vi "15-12-13 UHR-Fleezers Control (host) - 15.2.1UCB Darwin.vi"() -> ()   [LabVIEW 2014] (continued)
    n2915 = Build Array(w4201, w4200) -> (w4199:dbl[][])
    n2916 = Bundle(w4053, w4052, w4002) -> (w4057:cluster{u32[], u32[], u32[]})  [unwired: 1 in]
    n2917 = Build Array(w4053, w4052, w4002) -> (w4297:u32[][])
    n2918 = for {
      tunnel: w4053 -> [w4445] mode=indexing
      n2919 = call "Smart Buffer (DBL) 1.vi"("new element [write]"=w4445, "mode"=T25."write") -> ()  [unwired: 4 in, 6 out]
    }
    n2920 = local read "APD Integration Time (s)"() -> (w4068:dbl)
    n2921 = To Double Precision Float(number=w4297) -> (double precision float=w4298:dbl[][])
    n2922 = feedback #7 "APD3"(w4002) -> (w4003:u32[])
    n2923 = feedback #8 "APD2"(w4052) -> (w4225:u32[])
    n2924 = feedback #9 "APD1"(w4053) -> (w4296:u32[])
    n2925 = Build Array (concatenate)(w4003, w4002) -> (w4001:u32[])
    n2926 = Build Array (concatenate)(w4225, w4052) -> (w4224:u32[])
    n2927 = Build Array (concatenate)(w4296, w4053) -> (w4293:u32[])
    n2928 = for {
      tunnel: w4052 -> [w4444] mode=indexing
      n2929 = call "Smart Buffer (DBL) 2.vi"("new element [write]"=w4444, "mode"=T25."write") -> ()  [unwired: 4 in, 6 out]
    }
    n2930 = Array Size(array=w4293) -> (size(s)=w4290:i32)
    n2931 = Array Size(array=w4053) -> (size(s)=w4292:i32)
    n2932 = Multiply(x=w4292, y="APD Ave N") -> (x*y=w4291:dbl)
    n2933 = Greater?(x=w4290, y=w4291) -> (0:w4294:bool)
    n2934 = Bundle("APD 1", "APD 2", "APD 3") -> (w4328:cluster{string, string, string})  [unwired: 1 out]
    n2935 = local read "Trap Sets"() -> (w4260:u32)
    n2936 = case shown="True" w4294 {
      tunnel: w4293 -> [w4701 w4710]
      tunnel: [w4701 w4708] -> w4267
      tunnel: w4291 -> [_ w4703]
      tunnel: w4290 -> [_ w4709]
      tunnel: w4224 -> [w4700 w4707]
      tunnel: [w4700 w4706] -> w4222
      tunnel: w4001 -> [w4699 w4705]
      tunnel: [w4699 w4702] -> w4069
      frame False {
      }
      frame True {
        n2937 = Subtract(x=w4709, y=w4703) -> (x-y=w4704:dbl)
        n2938 = Array Subset "APD3"(array=w4705, index=w4704, length=w4703) -> (w4702:u32[])
        n2939 = Array Subset "APD2"(array=w4707, index=w4704, length=w4703) -> (w4706:u32[])
        n2940 = Array Subset "APD1"(array=w4710, index=w4704, length=w4703) -> (w4708:u32[])
      }
    }
    n2941 = feedback-in #7(w4069) -> ()
    n2942 = feedback-in #8(w4222) -> ()
    n2943 = feedback-in #9(w4267) -> ()
    n2944 = Cluster To Array(cluster=w4328) -> (array=w4325:string[])
    n2945 = for "APD" {
      tunnel: w4298 -> [w4970] mode=indexing
      tunnel: w4068 -> [w4977]
      tunnel: [w4973] -> w4226 mode=indexing
      tunnel: "APD Disp. Scale" -> [w4974]
      tunnel: w4325 -> [w4972] mode=indexing
      tunnel: "APD Disp. Downsample" -> [w4968]
      tunnel: [w4971] -> w4324
      workers-P: _ -> [_]
      tunnel: w4195 -> [w4967]
      n2946 = call "integrate 1D array interval - double.vi"("Ave N"=w4968, "Array In"=w4970) -> ("Array Out"=w4969:dbl[])  [unwired: 1 out]
      n2947 = Multiply(x=w4977, y=w4968) -> (x*y=w4971:dbl)
      n2948 = Divide(x=w4969, y=w4974) -> (x/y=w4975:dbl[])
      n2949 = Bundle By Name("t0"=w4967, "Y"=w4975, "dt"=w4971) -> (w4976:waveform(dbl))  [unwired: 1 out]
      n2950 = Set Waveform Attribute(5:w4972, 6:"NI_ChannelName" ("name"), 7:w4976) -> (3:w4973:waveform(dbl))  [unwired: 1 in, 2 out]
    }
    "APD Display Period (s)" <- w4324
    n2951 = Reciprocal(x=w4324) -> (1/x=→"APD Display Freq. (Hz)":dbl)
    n2952 = case "Deinterlace trap data, average down PSD" shown="2" w4260 {
      tunnel: w4168 -> [w4995 w5060]
      tunnel: [w4992 w5057] -> w4255
      tunnel: [w4995 w5059] -> w4159
      tunnel: "Detector Type" -> [w4994 w5055]
      tunnel: [w4993 w5058] -> w4254
      tunnel: [w4991 w5056] -> w4332
      frame 1, Default {
        n2953 = Divide(x=w4995, y=3276.7) -> (x/y=w4996:dbl[])
        n2954 = Decimate 1D Array(w4996) -> (w5005:dbl[], w5004:dbl[], w5003:dbl[], w5002:dbl[], w5001:dbl[], w5000:dbl[], w4999:dbl[], w4998:dbl[])
        n2955 = case shown="\"IR-QPD + PSD + FB-QPD position\"" w4994 {
          tunnel: w5005 -> [w5029 w5054]
          tunnel: w5004 -> [w5028 w5053]
          tunnel: w5003 -> [w5013 w5031]
          tunnel: w5002 -> [w5014 w5041]
          tunnel: w5001 -> [w5027 w5052]
          tunnel: w5000 -> [w5026 w5051]
          tunnel: w4999 -> [w5010 w5032]
          tunnel: w4998 -> [w5009 w5030]
          tunnel: [w5008 w5038] -> w4993
          tunnel: [w5007 w5037] -> w4992
          tunnel: [w5006 w5036] -> w4991
          frame "IR-QPD + PSD + FB-QPD", Default {
            w5006 = 0  # Channel pattern
            n2956 = Divide(x=w5029, y=w5014) -> (x/y=w5016:dbl[])
            n2957 = Divide(x=w5028, y=w5014) -> (x/y=w5015:dbl[])
            n2958 = Divide(x=w5027, y=w5010) -> (x/y=w5012:dbl[])
            n2959 = Divide(x=w5026, y=w5009) -> (x/y=w5011:dbl[])
            n2960 = Build Array(w5016, w5015, w5014, w5013, w5012, w5011, w5010, w5009) -> (w5007:dbl[][])
            n2961 = Bundle("T1 Y", "T1 X", "T1 Sum", "FB Sum", "PSD Y", "PSD X", "PSD Y Sum", "PSD X Sum") -> (w5025:T49)  [unwired: 1 out]
            n2962 = Cluster To Array(cluster=w5025) -> (array=w5008:string[])
          }
          frame "IR-QPD + PSD + FB-QPD position" {
            w5036 = 3  # Channel pattern
            n2963 = Negate(x=w5032) -> (-x=w5033:dbl[])
            n2964 = Divide(x=w5054, y=w5041) -> (x/y=w5043:dbl[])
            n2965 = Divide(x=w5053, y=w5041) -> (x/y=w5042:dbl[])
            n2966 = Divide(x=w5052, y=w5032) -> (x/y=w5040:dbl[])
            n2967 = Divide(x=w5051, y=w5033) -> (x/y=w5039:dbl[])
            n2968 = Build Array(w5043, w5042, w5041, w5030, w5031, w5040, w5039, w5032) -> (w5037:dbl[][])
            n2969 = Bundle("T1 Y", "T1 X", "T1 Sum", "FB X", "FB Sum", "PSD Y", "PSD X", "PSD Y Sum") -> (w5050:T49)  [unwired: 1 out]
            n2970 = Cluster To Array(cluster=w5050) -> (array=w5038:string[])
          }
        }
      }
      frame 2 {
        n2971 = case shown="\"IR-QPD + PSD + FB-QPD X position\", Default" w5055 {
          tunnel: w5060 -> [w5122 w5194 w5265]
          tunnel: [w5061 w5185 w5196] -> w5059
          tunnel: [w5088 w5176 w5243] -> w5058
          tunnel: [w5087 w5139 w5210] -> w5057
          tunnel: [w5081 w5174 w5241] -> w5056
          frame "IR-QPD + PSD + FB-QPD" {
            w5081 = 1  # Channel pattern
            # "time average x2 the 4th signal and the 4 psd signals (detection laser)"
            # "deinterlace 3 signals from qpd"
            n2972 = Decimate 1D Array(w5122) -> (w5121:i16[], w5120:i16[], w5086:i16[], w5119:i16[], w5109:i16[], w5107:i16[], w5106:i16[], w5104:i16[])
            n2973 = Decimate 1D Array(w5086) -> (w5085:i16[], w5084:i16[])
            n2974 = Decimate 1D Array(w5121) -> (w5118:i16[], w5090:i16[])
            n2975 = Decimate 1D Array(w5120) -> (w5117:i16[], w5115:i16[])
            n2976 = Decimate 1D Array(w5119) -> (w5116:i16[], w5114:i16[])
            n2977 = call "downsample 1D array - double.vi"("Ave N"=2.0, "Array In"=w5109) -> ("Array Out"=w5108:dbl[])  [unwired: 1 out]
            n2978 = call "downsample 1D array - double.vi"("Ave N"=2.0, "Array In"=w5107) -> ("Array Out"=w5089:dbl[])  [unwired: 1 out]
            n2979 = call "downsample 1D array - double.vi"("Ave N"=2.0, "Array In"=w5106) -> ("Array Out"=w5105:dbl[])  [unwired: 1 out]
            n2980 = call "downsample 1D array - double.vi"("Ave N"=2.0, "Array In"=w5104) -> ("Array Out"=w5103:dbl[])  [unwired: 1 out]
            n2981 = Interleave 1D Arrays(w5118, w5117, w5116, w5090, w5115, w5114, w5085, w5084, w5108, w5089, w5105, w5103) -> (w5102:dbl[])
            n2982 = Divide(x=w5102, y=3276.7) -> (x/y=w5101:dbl[])
            n2983 = Decimate 1D Array(w5101) -> (w5100:dbl[], w5099:dbl[], w5098:dbl[], w5097:dbl[], w5096:dbl[], w5095:dbl[], w5083:dbl[], w5082:dbl[], w5094:dbl[], w5093:dbl[], w5092:dbl[], w5091:dbl[])
            n2984 = Divide(x=w5100, y=w5098) -> (x/y=w5068:dbl[])
            n2985 = Divide(x=w5099, y=w5098) -> (x/y=w5067:dbl[])
            n2986 = Divide(x=w5097, y=w5095) -> (x/y=w5066:dbl[])
            n2987 = Divide(x=w5096, y=w5095) -> (x/y=w5065:dbl[])
            n2988 = Divide(x=w5094, y=w5092) -> (x/y=w5064:dbl[])
            n2989 = Divide(x=w5093, y=w5091) -> (x/y=w5063:dbl[])
            n2990 = Build Array(w5068, w5067, w5098, w5066, w5065, w5095, w5083, w5082, w5064, w5063, w5092, w5091) -> (w5087:dbl[][])
            n2991 = Bundle("T1 Y", "T1 X", "T1 Sum", "T2 Y", "T2 X", "T2 Sum", "T1 FB Sum", "T2 FB Sum", "PSD Y", "PSD X", "PSD Y Sum", "PSD X Sum") -> (w5069:T50)  [unwired: 1 out]
            n2992 = To Word Integer(number=w5102) -> (16bit integer=w5061:i16[])
            n2993 = Cluster To Array(cluster=w5069) -> (array=w5088:string[])
          }
          frame "IR-QPD + PSD + FB-QPD X position", Default {
            w5174 = 2  # Channel pattern
            # "time average x2 the 3 psd signals (detection laser)"
            # "deinterlace 3 signals from qpds"
            n2994 = Decimate 1D Array(w5194) -> (w5193:i16[], w5192:i16[], w5175:i16[], w5191:i16[], w5137:i16[], w5134:i16[], w5131:i16[], w5162:i16[])
            n2995 = Select(t=i16 -1, s="Flip X Sign", f=i16 1) -> (s? t:f=w5127:i16)
            n2996 = Multiply(x=w5192, y=w5127) -> (x*y=w5128:i16[])
            n2997 = Decimate 1D Array(w5175) -> (w5160:i16[], w5158:i16[])
            n2998 = Decimate 1D Array(w5193) -> (w5190:i16[], w5177:i16[])
            n2999 = Decimate 1D Array(w5128) -> (w5189:i16[], w5187:i16[])
            n3000 = Decimate 1D Array(w5191) -> (w5188:i16[], w5186:i16[])
            n3001 = Decimate 1D Array(w5162) -> (w5161:i16[], w5159:i16[])
            n3002 = call "downsample 1D array - I16.vi"("Ave N"=2.0, "Array In"=w5137) -> ("Array Out"=w5135:i16[])  [unwired: 1 in]
            n3003 = call "downsample 1D array - I16.vi"("Ave N"=2.0, "Array In"=w5131) -> ("Array Out"=w5129:i16[])  [unwired: 1 in]
            n3004 = call "downsample 1D array - I16.vi"("Ave N"=2.0, "Array In"=w5134) -> ("Array Out"=w5132:i16[])  [unwired: 1 in]
            n3005 = Interleave 1D Arrays(w5190, w5189, w5188, w5177, w5187, w5186, w5161, w5160, w5159, w5158, w5135, w5132, w5129) -> (w5185:i16[])
            n3006 = Divide(x=w5185, y=3276.7) -> (x/y=w5184:dbl[])
            n3007 = Decimate 1D Array(w5184) -> (w5183:dbl[], w5182:dbl[], w5181:dbl[], w5180:dbl[], w5179:dbl[], w5178:dbl[], w5150:dbl[], w5148:dbl[], w5147:dbl[], w5145:dbl[], w5144:dbl[], w5143:dbl[], w5140:dbl[])
            n3008 = Negate(x=w5140) -> (-x=w5138:dbl[])
            n3009 = Divide(x=w5144, y=w5140) -> (x/y=w5142:dbl[])
            n3010 = Divide(x=w5143, y=w5138) -> (x/y=w5141:dbl[])
            n3011 = Divide(x=w5183, y=w5181) -> (x/y=w5166:dbl[])
            n3012 = Divide(x=w5182, y=w5181) -> (x/y=w5165:dbl[])
            n3013 = Divide(x=w5180, y=w5178) -> (x/y=w5164:dbl[])
            n3014 = Divide(x=w5179, y=w5178) -> (x/y=w5163:dbl[])
            n3015 = Divide(x=w5150, y=w5148) -> (x/y=w5149:dbl[])
            n3016 = Divide(x=w5147, y=w5145) -> (x/y=w5146:dbl[])
            n3017 = Build Array(w5166, w5165, w5181, w5164, w5163, w5178, w5149, w5148, w5146, w5145, w5142, w5141, w5140) -> (w5139:dbl[][])
            n3018 = Bundle("T1 Y", "T1 X", "T1 Sum", "T2 Y", "T2 X", "T2 Sum", "T1 FB X", "T1 FB Sum", "T2 FB X", "T2 FB Sum", "PSD Y", "PSD X", "PSD Y Sum") -> (w5167:T51)  [unwired: 1 out]
            n3019 = Cluster To Array(cluster=w5167) -> (array=w5176:string[])
          }
          frame "IR-QPD + PSD + FB-QPD XY positions" {
            w5241 = 4  # Channel pattern
            # "time average x2 the 3 psd signals (detection laser)"
            # "deinterlace 3 signals from qpds"
            n3020 = Decimate 1D Array(w5265) -> (w5264:i16[], w5263:i16[], w5242:i16[], w5262:i16[], w5208:i16[], w5254:i16[], w5253:i16[], w5230:i16[])
            n3021 = Decimate 1D Array "Feedback Sum"(w5242) -> (w5226:i16[], w5224:i16[])
            n3022 = Decimate 1D Array "QPD Y"(w5264) -> (w5261:i16[], w5244:i16[])
            n3023 = Decimate 1D Array "QPD X"(w5263) -> (w5260:i16[], w5258:i16[])
            n3024 = Decimate 1D Array "Feedback Y"(w5208) -> (w5207:i16[], w5206:i16[])
            n3025 = Decimate 1D Array "QPD Sum"(w5262) -> (w5259:i16[], w5257:i16[])
            n3026 = Decimate 1D Array "Feedback X"(w5230) -> (w5227:i16[], w5225:i16[])
            n3027 = call "downsample 1D array - double.vi"("Ave N"=2.0, "Array In"=w5254) -> ("Array Out"=w5229:dbl[])  [unwired: 1 out]
            n3028 = call "downsample 1D array - double.vi"("Ave N"=2.0, "Array In"=w5253) -> ("Array Out"=w5228:dbl[])  [unwired: 1 out]
            n3029 = Interleave 1D Arrays(w5261, w5260, w5259, w5244, w5258, w5257, w5207, w5227, w5226, w5206, w5225, w5224, w5229, w5228) -> (w5252:dbl[])
            n3030 = Divide(x=w5252, y=3276.7) -> (x/y=w5251:dbl[])
            n3031 = Decimate 1D Array(w5251) -> (w5250:dbl[], w5249:dbl[], w5248:dbl[], w5247:dbl[], w5246:dbl[], w5245:dbl[], w5203:dbl[], w5217:dbl[], w5201:dbl[], w5202:dbl[], w5215:dbl[], w5199:dbl[], w5213:dbl[], w5211:dbl[])
            n3032 = Negate(x=w5211) -> (-x=w5209:dbl[])
            n3033 = Divide(x=w5213, y=w5209) -> (x/y=w5212:dbl[])
            n3034 = Divide(x=w5202, y=w5199) -> (x/y=w5198:dbl[])
            n3035 = Divide(x=w5203, y=w5201) -> (x/y=w5200:dbl[])
            n3036 = Divide(x=w5250, y=w5248) -> (x/y=w5234:dbl[])
            n3037 = Divide(x=w5249, y=w5248) -> (x/y=w5233:dbl[])
            n3038 = Divide(x=w5247, y=w5245) -> (x/y=w5232:dbl[])
            n3039 = Divide(x=w5246, y=w5245) -> (x/y=w5231:dbl[])
            n3040 = Divide(x=w5217, y=w5201) -> (x/y=w5216:dbl[])
            n3041 = Divide(x=w5215, y=w5199) -> (x/y=w5214:dbl[])
            n3042 = Build Array(w5234, w5233, w5248, w5232, w5231, w5245, w5200, w5216, w5201, w5198, w5214, w5199, w5212, w5211) -> (w5210:dbl[][])
            n3043 = Bundle("T1 Y", "T1 X", "T1 Sum", "T2 Y", "T2 X", "T2 Sum", "T1 FB Y", "T1 FB X", "T1 FB Sum", "T2 FB Y", "T2 FB X", "T2 FB Sum", "PSD X", "PSD Y Sum") -> (w5197:T52)  [unwired: 1 out]
            n3044 = To Word Integer(number=w5252) -> (16bit integer=w5196:i16[])
            n3045 = Cluster To Array(cluster=w5197) -> (array=w5243:string[])
          }
        }
      }
    }
    "AI labels" <- w4254
    n3046 = local read "APD Integration Time (s)"() -> (w4231:dbl)
    n3047 = Array Size(array=w4267) -> (size(s)=w4289:i32)
    n3048 = call <vilib>:"Std Deviation and Variance.vi"("X"=w4222) -> ("standard deviation"=w4221:dbl)  [unwired: 1 in, 2 out]
    n3049 = Add Array Elements(numeric array=w4222) -> (sum=w4223:u32)
    n3050 = Add Array Elements(numeric array=w4267) -> (sum=w4299:u32)
    n3051 = call <vilib>:"Std Deviation and Variance.vi"("X"=w4267) -> ("standard deviation"=w4266:dbl)  [unwired: 1 in, 2 out]
    n3052 = Divide(x=w4221, y=w4068) -> (x/y=w4218:dbl)
    "Rate sigma (Hz) 2" <- w4218
    n3053 = Multiply(x=w4068, y=w4289) -> (x*y=w4070:dbl)
    "Int. Time (s)" <- w4070
    n3054 = Divide(x=w4223, y=w4070) -> (x/y=w4219:dbl)
    "APD 2 Rate (Hz)" <- w4219
    n3055 = Multiply(x="APD Disp. Scale", y=w4226) -> (x*y=w4233:waveform(dbl)[])
    n3056 = Divide(x=w4299, y=w4070) -> (x/y=w4264:dbl)
    "APD 1 Rate (Hz)" <- w4264
    n3057 = Divide(x=w4266, y=w4068) -> (x/y=w4265:dbl)
    "Rate sigma (Hz)" <- w4265
    n3058 = Divide(x=w4218, y=w4219) -> (x/y=→"Sigma/Mean 2":dbl)
    n3059 = Multiply(x="APD Disp. Downsample", y=w4231) -> (x*y=w4229:dbl)
    n3060 = Divide(x=w4265, y=w4264) -> (x/y=→"Sigma/Mean":dbl)
    n3061 = Divide(x=w4233, y=w4229) -> (x/y=w4060:waveform(dbl)[])
    n3062 = Index Array(array=w4060, index=0) -> (element=w4215:waveform(dbl))
    n3063 = Index Array(array=w4060, index=1) -> (element=w4213:waveform(dbl))
    n3064 = Index Array(array=w4060, index=2) -> (element=w4062:waveform(dbl))
    n3065 = Subtract(x=w4215, y="APD 1 Offset") -> (x-y=w4211:waveform(dbl))
    n3066 = Subtract(x=w4213, y="APD 2 Offset") -> (x-y=w4210:waveform(dbl))
    n3067 = Subtract(x=w4062, y="APD 3 Offset") -> (x-y=w4059:waveform(dbl))
    n3068 = Add Array Elements(numeric array=w4069) -> (sum=w4072:u32)
    n3069 = call <vilib>:"Std Deviation and Variance.vi"("X"=w4069) -> ("standard deviation"=w4071:dbl)  [unwired: 1 in, 2 out]
    n3070 = Build Array(w4211, w4210, w4059) -> (→"APD Chart":waveform(dbl)[])
    n3071 = Divide(x=w4072, y=w4070) -> (x/y=w4066:dbl)
    "APD 3 Rate (Hz)" <- w4066
    n3072 = Divide(x=w4071, y=w4068) -> (x/y=w4067:dbl)
    "Rate sigma (Hz) 3" <- w4067
    n3073 = Divide(x=w4067, y=w4066) -> (x/y=→"Sigma/Mean 3":dbl)
    n3074 = local read "Data Period (s)"() -> (w4118:dbl)
    n3075 = local read "BD 1 Frequency 2 (MHz)"() -> (w4151:dbl)
    n3076 = local read "BD 1 Frequency 1 (MHz)"() -> (w4152:dbl)
    n3077 = Decimate 1D Array(w4159) -> (w4183:i16[], w4182:i16[], w4180:i16[], w4179:i16[])  [unwired: 9 out]
    n3078 = Multiply(x=w4118, y="Trap Pos. Disp. Downsample") -> (x*y=w4116:dbl)
    n3079 = Divide(x=w4183, y=w4182) -> (x/y=w4184:dbl[])
    n3080 = Divide(x=w4180, y=w4179) -> (x/y=w4181:dbl[])
    n3081 = local read "AOM X Cal (nm/MHz)"() -> (w4149:dbl)
    n3082 = Split 1D Array(array=w4184, index="N El. to Ave.") -> (second subarray=w4187:dbl[])  [unwired: 1 out]
    n3083 = Split 1D Array(array=w4181, index="N El. to Ave.") -> (second subarray=w4186:dbl[])  [unwired: 1 out]
    n3084 = Multiply(x=w4118, y="Trap Disp. Downsample") -> (x*y=w4197:dbl)
    "Display Period (s)" <- w4197
    n3085 = for "Trap AI" {
      tunnel: [w4990] -> w4026 mode=indexing
      tunnel: w4195 -> [w4981]
      tunnel: "Trap Disp. Downsample" -> [w4988]
      tunnel: w4255 -> [w4986] mode=indexing
      tunnel: w4118 -> [w4985]
      tunnel: w4254 -> [w4984] mode=indexing
      tunnel: [w4983] -> w4228 mode=indexing
      tunnel: w4197 -> [w4982]
      workers-P: _ -> [_]
      n3086 = Bundle By Name("Y"=w4986, "dt"=w4985) -> (w4987:waveform(dbl))  [unwired: 1 out]
      n3087 = Set Waveform Attribute(5:w4984, 6:"NI_ChannelName" ("name"), 7:w4987) -> (3:w4983:waveform(dbl))  [unwired: 1 in, 2 out]
      n3088 = call "downsample 1D array - double.vi"("Ave N"=w4988, "Array In"=w4986) -> ("Array Out"=w4989:dbl[])  [unwired: 1 out]
      n3089 = Bundle By Name(cluster=w4983, "t0"=w4981, "Y"=w4989, "dt"=w4982) -> (w4990:waveform(dbl))
    }
    n3090 = Bundle("BD 1 Frequency 1 (MHz)"=w4152, "BD 1 Frequency 2 (MHz)"=w4151) -> (w4153:T53)  [unwired: 1 out]
    n3091 = call-poly <vilib>:"Mean.vi"("X"=w4186) -> ("mean"=w4174:dbl)  [unwired: 1 out]
    n3092 = call-poly <vilib>:"Mean.vi"("X"=w4187) -> ("mean"=w4175:dbl)  [unwired: 1 out]
    n3093 = Reciprocal(x=w4197) -> (1/x=→"Trap Disp. Freq. (Hz)":dbl)
    n3094 = Cluster To Array(cluster=w4153) -> (array=w4150:dbl[])
    n3095 = local read "Trap X AI1 (DMA)"() -> (w4185:T15)
    n3096 = local read "Data points/scans (MCL)"() -> (w4309:dbl)
    n3097 = To Fixed-Point(number=w4174) -> (fixed-point=w4172:fxp<+/-,16,1>)  [unwired: 1 in]
    n3098 = To Fixed-Point(number=w4175) -> (fixed-point=w4173:fxp<+/-,16,1>)  [unwired: 1 in]
    n3099 = Bundle("Trap 1 Pos.", "Trap 2 Pos.") -> (w4194:cluster{string, string})  [unwired: 1 out]
    n3100 = Bundle By Name(cluster=w4185, "Set 1"=w4173, "Set 2"=w4172) -> (→"Trap X AI1 (DMA)":T15)
    n3101 = Cluster To Array(cluster=w4194) -> (array=w4191:string[])
    n3102 = Unbundle(w4057) -> (w4058:u32[])  [unwired: 2 out]
    n3103 = Select(t=-1.0, s="Negate Y Axis", f=1.0) -> (s? t:f=w4135:dbl)
    n3104 = for "Trap Position" {
      tunnel: w4199 -> [w4615] mode=indexing
      tunnel: "Trap Pos. Disp. Downsample" -> [w4614]
      tunnel: w4116 -> [w4612]
      tunnel: w4195 -> [w4611]
      tunnel: w4191 -> [w4609] mode=indexing
      tunnel: [w4608] -> w4105 mode=indexing
      tunnel: w4150 -> [w4606] mode=indexing
      tunnel: w4149 -> [w4604]
      tunnel: w4135 -> [w4603]
      n3105 = call "downsample 1D array - double.vi"("Ave N"=w4614, "Array In"=w4615) -> ("Array Out"=w4613:dbl[])  [unwired: 1 out]
      n3106 = Subtract(x=w4613, y=w4606) -> (x-y=w4607:dbl[])
      n3107 = Multiply(x=w4604, y=w4607) -> (x*y=w4605:dbl[])
      n3108 = Multiply(x=w4603, y=w4605) -> (x*y=w4602:dbl[])
      n3109 = Bundle By Name("Y"=w4602, "dt"=w4612, "t0"=w4611) -> (w4610:waveform(dbl))  [unwired: 1 out]
      n3110 = Set Waveform Attribute(5:w4609, 6:"NI_ChannelName" ("name"), 7:w4610) -> (3:w4608:waveform(dbl))  [unwired: 1 in, 2 out]
    }
    n3111 = To Double Precision Float(number=w4058) -> (double precision float=w4252:dbl[])
    n3112 = local read "Display Period (s)"() -> (w4243:dbl)
    n3113 = Increment(x=w4309) -> (x+1=w4310:dbl)
    n3114 = Index Array(array=w4105, index=0) -> (element=w4109:waveform(dbl))
    n3115 = Index Array(array=w4105, index=1) -> (element=w4104:waveform(dbl))
    n3116 = feedback #10(w4310) -> (w4313:dbl)
    n3117 = Select(t=0, s=w4300, f=w4313) -> (s? t:f=w4306:dbl)
    n3118 = Array Size(array=w4252) -> (size(s)=w4312:i32)
    n3119 = Add(x=w4312, y=w4306) -> (x+y=w4307:dbl)
    n3120 = Unbundle By Name(w4109) -> ("Y"=w4110:dbl[])
    n3121 = Divide(x="Bead Sep. Int. Time (s)", y=w4243) -> (x/y=w4145:dbl)
    n3122 = Add(x=w4110, y="FB Trap Pos Offset") -> (x+y=w4108:dbl[])
    "T1 x pos data" <- w4108
    n3123 = Greater?(x=w4307, y=w4309) -> (0:w4308:bool)
    n3124 = feedback #11(w4108) -> (w4147:dbl[])
    n3125 = Build Array (concatenate)(w4108, w4147) -> (w4146:dbl[])
    n3126 = Bundle By Name(cluster=w4109, "Y"=w4108) -> (w4107:waveform(dbl))
    n3127 = Select(t=w4306, s=w4308, f=w4307) -> (s? t:f=w4305:dbl)
    n3128 = feedback-in #10(w4305) -> ()
    n3129 = local read "MCL Scanning"() -> (w4303:bool)
    n3130 = Bundle(w4107, w4104) -> (w4103:cluster{waveform(dbl), waveform(dbl)})  [unwired: 1 out]
    n3131 = Index Array(array=w4026, index="index 1") -> (element=w4047:waveform(dbl))
    n3132 = Index Array(array=w4026, index="index 2") -> (element=w4051:waveform(dbl))
    n3133 = Split 1D Array(array=w4146, index=w4145) -> (first subarray=w4139:dbl[])  [unwired: 1 out]
    n3134 = feedback-in #11(w4139) -> ()
    n3135 = Unbundle By Name(w4047) -> ("Y"=w4046:dbl[])
    n3136 = Unbundle By Name(w4051) -> ("Y"=w4050:dbl[])
    n3137 = Not(x=w4308) -> (.not. x?=w4302:bool)
    n3138 = Cluster To Array(cluster=w4103) -> (array=w4082:waveform(dbl)[])
    "Trap Positions" <- w4082
    n3139 = call-poly <vilib>:"Mean.vi"("X"=w4139) -> ("mean"=w4138:dbl)  [unwired: 1 out]
    "Mean T1 Position (nm)" <- w4138
    n3140 = Subtract(x=w4139, y=w4138) -> (x-y=w4144:dbl[])
    n3141 = Square(x=w4144) -> (x^2=w4143:dbl[])
    n3142 = And(x=w4302, y=w4303) -> (x .and. y?=w4304:bool)
    n3143 = call-poly <vilib>:"Mean.vi"("X"=w4143) -> ("mean"=w4142:dbl)  [unwired: 1 out]
    n3144 = call-poly <vilib>:"Mean.vi"("X"=w4046) -> ("mean"=→"Trap 1 sum mean":dbl)  [unwired: 1 out]
    n3145 = call-poly <vilib>:"Mean.vi"("X"=w4050) -> ("mean"=→"Trap 2 sum mean":dbl)  [unwired: 1 out]
    n3146 = Square Root(x=w4142) -> (sqrt(x)=w4141:dbl)
    n3147 = Or(x=w4304, y=w4300) -> (x .or. y?=w4301:bool)
    n3148 = Build Array (concatenate)(w4226, w4026) -> (w4006:waveform(dbl)[])
    "All Signals" <- w4006
    n3149 = Equal?(x="Tab Control 6", y=T43."High Res Display") -> (x = y?=w4256:bool)
    n3150 = case shown="False" "X or Y?" {
      tunnel: w4026 -> [w4434 w4440]
      tunnel: [w4435 w4439] -> w4021
      tunnel: [w4433 w4438] -> w4018
      frame False {
        n3151 = Index Array(array=w4434, index=0) -> (element=w4435:waveform(dbl))
        n3152 = Index Array(array=w4434, index=3) -> (element=w4433:waveform(dbl))
      }
      frame True {
        n3153 = Index Array(array=w4440, index=1) -> (element=w4439:waveform(dbl))
        n3154 = Index Array(array=w4440, index=4) -> (element=w4438:waveform(dbl))
      }
    }
    n3155 = Multiply(x=10.0, y=w4141) -> (x*y=→"Trap 1 Position RMS (A)":dbl)
    n3156 = case "For displaying the high resolution display (no downsampling)" shown="True" w4256 {
      tunnel: w4228 -> [_ w4635]
      frame False {
      }
      frame True {
        n3157 = Index Array(array=w4635, index="High Res. Display") -> (element=w4636:waveform(dbl))
        n3158 = call <vilib>:"Std Deviation and Variance.vi"("X"=w4636) -> ("mean"=w4643:dbl, "standard deviation"=w4648:dbl)  [unwired: 1 in, 1 out]
        "Mean Intensity" <- w4643
        "Sigma" <- w4648
        n3159 = Subtract(x=w4636, y=w4643) -> (x-y=w4642:waveform(dbl))
        n3160 = Select(t=w4642, s="Subtract mean", f=w4636) -> (s? t:f=→"1 Channel":waveform(dbl))
        n3161 = Divide(x=w4648, y=w4643) -> (x/y=→"Sigma/Mean":dbl)
        n3162 = feedback #12(1) -> (w4637:i32)
        n3163 = Greater Or Equal?(x=w4637, y="Slow mean N ave.") -> (x >= y?=w4650:bool)
        n3164 = Increment(x=w4637) -> (x+1=w4652:i32)
        n3165 = Select(t=1, s=w4650, f=w4652) -> (s? t:f=w4639:i32)
        n3166 = feedback-in #12(w4639) -> ()
        n3167 = feedback #13() -> (w4640:waveform(dbl))  [unwired: 1 out]
        n3168 = case shown="Default" w4637 {
          tunnel: [w4655 w4658] -> w4641
          tunnel: w4640 -> [w4657 _]
          tunnel: w4636 -> [w4656 w4658]
          frame Default {
            n3169 = call-poly <vilib>:"Append Waveforms.vi"("waveform B"=w4656, "waveform A"=w4657) -> ("waveform out"=w4655:waveform(dbl))  [unwired: 1 in, 8 out]
          }
          frame 1 {
          }
        }
        n3170 = feedback-in #13(w4641) -> ()
        n3171 = case shown="True" w4650 {
          tunnel: w4641 -> [_ w4654]
          frame False {
          }
          frame True {
            n3172 = call-poly <vilib>:"Mean.vi"("X"=w4654) -> ("mean"=→"Slow mean":dbl)  [unwired: 1 out]
          }
        }
      }
    }
    n3173 = case "For plotting results of scanning MCL (fluorescence and detection laser images)" shown="True" w4301 {
      tunnel: w4300 -> [_ w4718]
      tunnel: w4309 -> [_ _]
      tunnel: w4228 -> [_ w4814]
      tunnel: w4208 -> [_ w4746]
      tunnel: w4057 -> [_ w4724]
      frame False {
      }
      frame True {
        n3174 = Unbundle(w4724) -> (w4723:u32[], w4721:u32[], w4719:u32[])
        n3175 = To Double Precision Float(number=w4723) -> (double precision float=w4722:dbl[])
        n3176 = To Double Precision Float(number=w4721) -> (double precision float=w4720:dbl[])
        n3177 = To Double Precision Float(number=w4719) -> (double precision float=w4712:dbl[])
        n3178 = Index Array(array=w4814, index=10) -> (element=w4820:waveform(dbl))
        n3179 = Index Array(array=w4814, index=11) -> (element=w4817:waveform(dbl))
        n3180 = local read "Cycles/step (MCL)"() -> (w4776:u64)
        n3181 = Index Array(array=w4814, index="Channel") -> (element=w4816:waveform(dbl))
        n3182 = Unbundle(w4746) -> ("New Image"=w4745:T2, "New Image"=w4744:T2, "New Image"=w4725:T2, "New Image"=w4726:T2, "New Image"=w4727:T2)
        n3183 = local read "Scan steps (MCL)"() -> (w4714:u64)
        n3184 = Unbundle By Name(w4820) -> ("Y"=w4778:dbl[])
        n3185 = Unbundle By Name(w4817) -> ("Y"=w4780:dbl[])
        n3186 = local read "Scan lines (y)"() -> (w4715:u64)
        n3187 = local read "N APD Samp/step"() -> (w4717:dbl)
        n3188 = Unbundle By Name(w4816) -> ("Y"=w4785:dbl[])
        n3189 = call "downsample 1D array - double.vi"("Ave N"=w4776, "Array In"=w4778) -> ("Array Out"=w4777:dbl[])  [unwired: 1 out]
        n3190 = call "downsample 1D array - double.vi"("Ave N"=w4776, "Array In"=w4780) -> ("Array Out"=w4779:dbl[])  [unwired: 1 out]
        n3191 = call "downsample 1D array - double.vi"("Ave N"=w4776, "Array In"=w4785) -> ("Array Out"=w4784:dbl[])  [unwired: 1 out]
        n3192 = Multiply(x=w4714, y=u64 2) -> (x*y=w4716:u64)
        n3193 = feedback #14(w4720) -> (w4764:dbl[])
        n3194 = Build Array (concatenate)(w4764, w4720) -> (w4763:dbl[])
        n3195 = feedback #15(w4712) -> (w4713:dbl[])
        n3196 = Build Array (concatenate)(w4713, w4712) -> (w4711:dbl[])
        n3197 = Select(t=w4720, s=w4718, f=w4763) -> (s? t:f=w4748:dbl[])
        n3198 = feedback-in #14(w4748) -> ()
        n3199 = Select(t=w4712, s=w4718, f=w4711) -> (s? t:f=w4729:dbl[])
        n3200 = feedback-in #15(w4729) -> ()
        n3201 = feedback #16(w4722) -> (w4839:dbl[])
        n3202 = Build Array (concatenate)(w4839, w4722) -> (w4822:dbl[])
        n3203 = Select(t=w4722, s=w4718, f=w4822) -> (s? t:f=w4826:dbl[])
        n3204 = feedback-in #16(w4826) -> ()
        n3205 = feedback #17(w4777) -> (w4828:dbl[])
        n3206 = Build Array (concatenate)(w4828, w4777) -> (w4819:dbl[])
        n3207 = feedback #18(w4784) -> (w4837:dbl[])
        n3208 = Build Array (concatenate)(w4837, w4784) -> (w4836:dbl[])
        n3209 = feedback #19(w4779) -> (w4830:dbl[])
        n3210 = Build Array (concatenate)(w4830, w4779) -> (w4831:dbl[])
        n3211 = Select(t=w4777, s=w4718, f=w4819) -> (s? t:f=w4781:dbl[])
        n3212 = feedback-in #17(w4781) -> ()
        n3213 = Select(t=w4784, s=w4718, f=w4836) -> (s? t:f=w4783:dbl[])
        n3214 = feedback-in #18(w4783) -> ()
        n3215 = Select(t=w4779, s=w4718, f=w4831) -> (s? t:f=w4782:dbl[])
        n3216 = feedback-in #19(w4782) -> ()
        n3217 = call "integrate 1D array interval - double.vi"("Ave N"=w4717, "Array In"=w4748) -> ("Array Out"=w4759:dbl[])  [unwired: 1 out]
        n3218 = call "integrate 1D array interval - double.vi"("Ave N"=w4717, "Array In"=w4729) -> ("Array Out"=w4740:dbl[])  [unwired: 1 out]
        n3219 = call "integrate 1D array interval - double.vi"("Ave N"=w4717, "Array In"=w4826) -> ("Array Out"=w4825:dbl[])  [unwired: 1 out]
        n3220 = Array Size(array=w4759) -> (size(s)=w4760:i32)
        n3221 = Array Size(array=w4740) -> (size(s)=w4741:i32)
        n3222 = Array Size(array=w4825) -> (size(s)=w4827:i32)
        n3223 = Multiply(x=w4715, y=w4716) -> (x*y=w4762:u64)
        n3224 = Multiply(x=w4715, y=w4716) -> (x*y=w4743:u64)
        n3225 = Multiply(x=w4715, y=w4716) -> (x*y=w4835:u64)
        n3226 = Subtract(x=w4762, y=w4760) -> (x-y=w4753:u64)
        n3227 = call-poly <vilib>:"Mean.vi"("X"=w4759) -> ("mean"=w4750:dbl)  [unwired: 1 out]
        n3228 = Subtract(x=w4743, y=w4741) -> (x-y=w4734:u64)
        n3229 = call-poly <vilib>:"Mean.vi"("X"=w4740) -> ("mean"=w4731:dbl)  [unwired: 1 out]
        n3230 = Subtract(x=w4835, y=w4827) -> (x-y=w4775:u64)
        n3231 = call-poly <vilib>:"Mean.vi"("X"=w4825) -> ("mean"=w4772:dbl)  [unwired: 1 out]
        n3232 = call-poly <vilib>:"Mean.vi"("X"=w4781) -> ("mean"=w4765:dbl)  [unwired: 1 out]
        n3233 = call-poly <vilib>:"Mean.vi"("X"=w4783) -> ("mean"=w4770:dbl)  [unwired: 1 out]
        n3234 = call-poly <vilib>:"Mean.vi"("X"=w4782) -> ("mean"=w4768:dbl)  [unwired: 1 out]
        n3235 = Initialize Array(1.0 ("element"), w4753) -> (w4749:dbl[])
        n3236 = Initialize Array(1.0 ("element"), w4734) -> (w4730:dbl[])
        n3237 = Initialize Array(1.0 ("element"), w4775) -> (w4766:dbl[])
        n3238 = Multiply(x=w4749, y=w4750) -> (x*y=w4751:dbl[])
        n3239 = Multiply(x=w4730, y=w4731) -> (x*y=w4732:dbl[])
        n3240 = Multiply(x=w4766, y=w4772) -> (x*y=w4773:dbl[])
        n3241 = Multiply(x=w4766, y=w4768) -> (x*y=w4769:dbl[])
        n3242 = Multiply(x=w4766, y=w4770) -> (x*y=w4771:dbl[])
        n3243 = Multiply(x=w4766, y=w4765) -> (x*y=w4767:dbl[])
        n3244 = Build Array (concatenate)(w4759, w4751) -> (w4761:dbl[])
        n3245 = Build Array (concatenate)(w4740, w4732) -> (w4742:dbl[])
        n3246 = Build Array (concatenate)(w4825, w4773) -> (w4834:dbl[])
        n3247 = Build Array (concatenate)(w4781, w4767) -> (w4829:dbl[])
        n3248 = Build Array (concatenate)(w4783, w4771) -> (w4833:dbl[])
        n3249 = Build Array (concatenate)(w4782, w4769) -> (w4832:dbl[])
        n3250 = Reshape Array(w4761, w4715, w4716) -> (w4757:dbl[][])
        n3251 = Reshape Array(w4742, w4715, w4716) -> (w4738:dbl[][])
        n3252 = Reshape Array(w4834, w4715, w4716) -> (w4812:dbl[][])
        n3253 = Reshape Array(w4829, w4715, w4716) -> (w4795:dbl[][])
        n3254 = Reshape Array(w4833, w4715, w4716) -> (w4787:dbl[][])
        n3255 = Reshape Array(w4832, w4715, w4716) -> (w4802:dbl[][])
        n3256 = Array Subset(array=w4757, index (col)=0 ("index"), length (col)=w4714) -> (w4756:dbl[][])  [unwired: 2 in]
        n3257 = Array Subset(array=w4757, index (col)=w4714) -> (w4754:dbl[][])  [unwired: 3 in]
        n3258 = Array Subset(array=w4738, index (col)=0 ("index"), length (col)=w4714) -> (w4737:dbl[][])  [unwired: 2 in]
        n3259 = Array Subset(array=w4738, index (col)=w4714) -> (w4735:dbl[][])  [unwired: 3 in]
        n3260 = Array Subset(array=w4802, index (col)=0 ("index"), length (col)=w4714) -> (w4807:dbl[][])  [unwired: 2 in]
        n3261 = Array Subset(array=w4802, index (col)=w4714) -> (w4805:dbl[][])  [unwired: 3 in]
        n3262 = Array Subset(array=w4812, index (col)=0 ("index"), length (col)=w4714) -> (w4811:dbl[][])  [unwired: 2 in]
        n3263 = Array Subset(array=w4812, index (col)=w4714) -> (w4809:dbl[][])  [unwired: 3 in]
        n3264 = Array Subset(array=w4787, index (col)=0 ("index"), length (col)=w4714) -> (w4793:dbl[][])  [unwired: 2 in]
        n3265 = Array Subset(array=w4787, index (col)=w4714) -> (w4791:dbl[][])  [unwired: 3 in]
        n3266 = Array Subset(array=w4795, index (col)=0 ("index"), length (col)=w4714) -> (w4800:dbl[][])  [unwired: 2 in]
        n3267 = Array Subset(array=w4795, index (col)=w4714) -> (w4798:dbl[][])  [unwired: 3 in]
        n3268 = for {
          tunnel: w4756 -> [w4888] mode=indexing
          tunnel: [w4887] -> w4755 mode=indexing
          workers-P: _ -> [_]
          n3269 = Reverse 1D Array(array=w4888) -> (reversed array=w4887:dbl[])
        }
        n3270 = for {
          tunnel: w4737 -> [w4886] mode=indexing
          tunnel: [w4885] -> w4736 mode=indexing
          workers-P: _ -> [_]
          n3271 = Reverse 1D Array(array=w4886) -> (reversed array=w4885:dbl[])
        }
        n3272 = for {
          tunnel: w4807 -> [w4894] mode=indexing
          tunnel: [w4893] -> w4806 mode=indexing
          workers-P: _ -> [_]
          n3273 = Reverse 1D Array(array=w4894) -> (reversed array=w4893:dbl[])
        }
        n3274 = for {
          tunnel: w4811 -> [w4896] mode=indexing
          tunnel: [w4895] -> w4810 mode=indexing
          workers-P: _ -> [_]
          n3275 = Reverse 1D Array(array=w4896) -> (reversed array=w4895:dbl[])
        }
        n3276 = for {
          tunnel: w4793 -> [w4890] mode=indexing
          tunnel: [w4889] -> w4792 mode=indexing
          workers-P: _ -> [_]
          n3277 = Reverse 1D Array(array=w4890) -> (reversed array=w4889:dbl[])
        }
        n3278 = for {
          tunnel: w4800 -> [w4892] mode=indexing
          tunnel: [w4891] -> w4799 mode=indexing
          workers-P: _ -> [_]
          n3279 = Reverse 1D Array(array=w4892) -> (reversed array=w4891:dbl[])
        }
        n3280 = Index Array(array=w4812, index (row)=0) -> (element=→"Waveform Graph":dbl[])  [unwired: 1 in]
        n3281 = Add(x=w4755, y=w4754) -> (x+y=w4747:dbl[][])
        n3282 = Add(x=w4736, y=w4735) -> (x+y=w4728:dbl[][])
        n3283 = Add(x=w4806, y=w4805) -> (x+y=w4804:dbl[][])
        n3284 = Add(x=w4810, y=w4809) -> (x+y=w4786:dbl[][])
        n3285 = Add(x=w4792, y=w4791) -> (x+y=w4790:dbl[][])
        n3286 = Add(x=w4799, y=w4798) -> (x+y=w4797:dbl[][])
        n3287 = Divide(x=w4790, y=2) -> (x/y=w4788:dbl[][])
        n3288 = disable-structure shown="Disabled" {
          disable-tunnel: w4804 -> [w4883 _]
          disable-tunnel: 2 -> [w4882 _]
          disable-tunnel: w4797 -> [w4881 _]
          disable-tunnel: 2 -> [w4880 _]
          disable-tunnel: w4788 -> [w4879 _]
          disable-tunnel: w4786 -> [w4876 _]
          disable-tunnel: w4747 -> [w4854 _]
          disable-tunnel: w4745 -> [w4852 _]
          disable-tunnel: w4744 -> [w4851 _]
          disable-tunnel: w4728 -> [w4844 _]
          disable-tunnel: w4727 -> [w4842 _]
          disable-tunnel: w4726 -> [w4841 _]
          disable-tunnel: w4725 -> [w4840 _]
          frame Disabled {
            w4849 = u32 0 items=["Horizontal", "Vertical", "Central", "1st Diagonal", "2nd Diagonal"] ("Type of Symmetry")
            w4859 = u32 0 items=["Horizontal", "Vertical", "Central", "1st Diagonal", "2nd Diagonal"] ("Type of Symmetry")
            w4866 = u32 0 items=["Horizontal", "Vertical", "Central", "1st Diagonal", "2nd Diagonal"] ("Type of Symmetry")
            w4869 = u32 0 items=["Horizontal", "Vertical", "Central", "1st Diagonal", "2nd Diagonal"] ("Type of Symmetry")
            w4877 = u32 0 items=["Horizontal", "Vertical", "Central", "1st Diagonal", "2nd Diagonal"] ("Type of Symmetry")
            n3289 = Divide(x=w4883, y=w4882) -> (x/y=w4862:dbl[][])
            n3290 = To Single Precision Float(number=w4876) -> (single precision float=w4875:sgl[][])
            n3291 = To Single Precision Float(number=w4854) -> (single precision float=w4858:sgl[][])
            n3292 = To Single Precision Float(number=w4844) -> (single precision float=w4848:sgl[][])
            n3293 = Divide(x=w4881, y=w4880) -> (x/y=w4864:dbl[][])
            n3294 = Transpose 2D Array(2D array=w4879) -> (transposed array=→"Data map":dbl[][])
            n3295 = To Single Precision Float(number=w4862) -> (single precision float=w4868:sgl[][])
            n3296 = To Single Precision Float(number=w4864) -> (single precision float=w4865:sgl[][])
            n3297 = call "IMAQ ArrayToImage"("Image Pixels (Float)"=w4875, "Image"=w4852) -> ("Image Out"=w4878:T2)  [unwired: 8 in, 1 out]
            n3298 = call "IMAQ ArrayToImage"("Image Pixels (Float)"=w4858, "Image"=w4851) -> ("Image Out"=w4860:T2)  [unwired: 8 in, 1 out]
            n3299 = call "IMAQ ArrayToImage"("Image Pixels (Float)"=w4848, "Image"=w4840) -> ("Image Out"=w4850:T2)  [unwired: 8 in, 1 out]
            n3300 = call "IMAQ ArrayToImage"("Image Pixels (Float)"=w4868, "Image"=w4841) -> ("Image Out"=w4870:T2)  [unwired: 8 in, 1 out]
            n3301 = call "IMAQ Symmetry"("Type of Symmetry"=w4877, "Image Src"=w4878) -> ("Image Dst Out"=w4873:T2)  [unwired: 3 in, 1 out]
            n3302 = call "IMAQ ArrayToImage"("Image Pixels (Float)"=w4865, "Image"=w4842) -> ("Image Out"=w4867:T2)  [unwired: 8 in, 1 out]
            n3303 = call "IMAQ Symmetry"("Type of Symmetry"=w4859, "Image Src"=w4860) -> ("Image Dst Out"=w4856:T2)  [unwired: 3 in, 1 out]
            n3304 = call "IMAQ Symmetry"("Type of Symmetry"=w4849, "Image Src"=w4850) -> ("Image Dst Out"=w4846:T2)  [unwired: 3 in, 1 out]
            n3305 = call "IMAQ Symmetry"("Type of Symmetry"=w4869, "Image Src"=w4870) -> ("Image Dst Out"=→"Detection Laser X":T2)  [unwired: 3 in, 1 out]
            n3306 = call "IMAQ Symmetry"("Type of Symmetry"=w4866, "Image Src"=w4867) -> ("Image Dst Out"=→"Detection Laser Y":T2)  [unwired: 3 in, 1 out]
            n3307 = call "IMAQ Set Simple Calibration"("Calibration Axis Info"=T44 {"Origin Pixel"={"X"=0.0, "Y"=0.0}, "Angle Relative to Horizontal (deg)"=0.0, "Axis Reference"=0}, "Grid Descriptor"=T45 {"X Step"=0.3, "Y Step"=0.3, "Unit"=enum."Undefined"}, "Image"=w4873) -> ("Calibrated Image"=→"APD 1":T2)  [unwired: 7 in, 1 out]
            n3308 = call "IMAQ Set Simple Calibration"("Calibration Axis Info"=T44 {"Origin Pixel"={"X"=0.0, "Y"=0.0}, "Angle Relative to Horizontal (deg)"=0.0, "Axis Reference"=0}, "Grid Descriptor"=T45 {"X Step"=0.3, "Y Step"=0.3, "Unit"=enum."Undefined"}, "Image"=w4856) -> ("Calibrated Image"=→"APD 2":T2)  [unwired: 7 in, 1 out]
            n3309 = call "IMAQ Set Simple Calibration"("Calibration Axis Info"=T44 {"Origin Pixel"={"X"=0.0, "Y"=0.0}, "Angle Relative to Horizontal (deg)"=0.0, "Axis Reference"=0}, "Grid Descriptor"=T45 {"X Step"=0.3, "Y Step"=0.3, "Unit"=enum."Undefined"}, "Image"=w4846) -> ("Calibrated Image"=→"APD 3":T2)  [unwired: 7 in, 1 out]
          }
          frame Enabled {
          }
        }
      }
    }
    n3310 = case "For computing FFTs for display" shown="True" "Compute FFT" {
      tunnel: w4228 -> [_ w5368]
      frame False {
      }
      frame True {
        n3311 = Build Array("FFT 1 Choice 1", "FFT 1 Choice 2", "FFT 2 Choice 1", "FFT 2 Choice 2") -> (w5361:u16[])
        n3312 = Array Size(array=w5368) -> (size(s)=w5367:i32)
        n3313 = feedback-in #20(w5361) -> ()
        n3314 = feedback #20(u16[] [100, 100, 100, 100]) -> (w5362:u16[])
        n3315 = feedback-in #21("# Spectra to Ave.") -> ()
        n3316 = feedback #21("# Spectra to Ave.") -> (w5359:dbl)
        n3317 = Not Equal?(x="# Spectra to Ave.", y=w5359) -> (x != y?=w5358:bool)
        n3318 = Not Equal?(x=w5361, y=w5362) -> (x != y?=w5360:bool)
        n3319 = feedback #22(1.0) -> (w5345:dbl)
        n3320 = Compound Arithmetic op=OR("Reset FFT", w5360, w5358) -> (w5343:bool)
        n3321 = Select(t=1.0, s=w5343, f=w5345) -> (s? t:f=w5347:dbl)
        n3322 = Greater?(x=w5347, y="# Spectra to Ave.") -> (0:w5366:bool)
        n3323 = Increment(x=w5347) -> (x+1=w5346:dbl)
        n3324 = feedback-in #22(w5346) -> ()
        n3325 = local read "DMA Update Period (s)"() -> (w5341:dbl)
        n3326 = Multiply(x="# Spectra to Ave.", y=w5341) -> (x*y=→"Ave. Time (s)":dbl)
        n3327 = Build Array(cluster{"f0":dbl, "df":dbl, "magnitude":dbl[]} {"f0"=0.0, "df"=0.0, "magnitude"=[]} ("PSD")) -> (w5350:cluster{"f0":dbl, "df":dbl, "magnitude":dbl[]}[])
        n3328 = Build Array(w5350, w5350, w5350, w5350) -> (w5352:T54)
        n3329 = feedback #23(w5352) -> (w5357:T54)
        n3330 = for {
          N: 4 -> [_]
          tunnel: w5361 -> [w5390] mode=indexing
          tunnel: w5368 -> [w5391]
          tunnel: w5367 -> [w5393]
          tunnel: w5343 -> [w5386]
          tunnel: w5366 -> [w5385]
          tunnel: "# Spectra to Ave." -> [w5384]
          tunnel: [w5383] -> w5356 mode=indexing
          tunnel: w5357 -> [w5388] mode=indexing
          tunnel: [w5387] -> w5344 mode=indexing
          tunnel: w5347 -> [w5382]
          n3331 = Less?(x=w5390, y=w5393) -> (x < y?=w5392:bool)
          n3332 = Index Array(array=w5391, index=w5390) -> (element=w5389:waveform(dbl))
          n3333 = case shown="True" w5392 {
            tunnel: w5389 -> [_ w5410]
            tunnel: w5388 -> [w5395 w5408]
            tunnel: [w5395 w5396] -> w5387
            tunnel: w5386 -> [_ w5407]
            tunnel: w5385 -> [_ w5400]
            tunnel: w5384 -> [_ w5399]
            tunnel: [cluster{"f0":dbl, "df":dbl, "magnitude":dbl[]} {"f0"=0.0, "df"=0.0, "magnitude"=[]} ("PSD") w5401] -> w5383
            tunnel: w5382 -> [_ w5398]
            frame False {
            }
            frame True {
              n3334 = call <vilib>:"Std Deviation and Variance.vi"("X"=w5410) -> ("mean"=w5411:dbl)  [unwired: 1 in, 2 out]
              n3335 = Subtract(x=w5410, y=w5411) -> (x-y=w5409:waveform(dbl))
              n3336 = xnode "Spectral Measurements"("Signals"=w5409) -> ("PSD"=w5403:cluster{"f0":dbl, "df":dbl, "magnitude":dbl[]})  [unwired: 1 in, 1 out]
              n3337 = case shown="False" w5407 {
                tunnel: w5408 -> [w5420 _]
                tunnel: [w5416 w5425] -> w5396
                tunnel: w5403 -> [w5419 w5426]
                tunnel: w5400 -> [w5418 _]
                frame False {
                  n3338 = Build Array (concatenate)(w5420, w5419) -> (w5417:cluster{"f0":dbl, "df":dbl, "magnitude":dbl[]}[])
                  n3339 = case shown="True" w5418 {
                    tunnel: w5417 -> [w5421 w5424]
                    tunnel: [w5421 w5422] -> w5416
                    frame False {
                    }
                    frame True {
                      n3340 = Delete From Array(array=w5424, index=0) -> (array with subset deleted=w5422:cluster{"f0":dbl, "df":dbl, "magnitude":dbl[]}[])  [unwired: 1 in, 1 out]
                    }
                  }
                }
                frame True {
                  n3341 = Build Array(w5426) -> (w5425:cluster{"f0":dbl, "df":dbl, "magnitude":dbl[]}[])
                }
              }
              n3342 = for {
                tunnel: w5396 -> [w5415] mode=indexing
                tunnel: [w5414] -> w5406 mode=indexing
                workers-P: _ -> [_]
                n3343 = Unbundle By Name(w5415) -> ("magnitude"=w5414:dbl[])
              }
              n3344 = Transpose 2D Array(2D array=w5406) -> (transposed array=w5405:dbl[][])
              n3345 = for {
                tunnel: w5405 -> [w5413] mode=indexing
                tunnel: [w5412] -> w5404 mode=indexing
                workers-P: _ -> [_]
                n3346 = Add Array Elements(numeric array=w5413) -> (sum=w5412:dbl)
              }
              n3347 = Select(t=w5399, s=w5400, f=w5398) -> (s? t:f=w5397:dbl)
              n3348 = Divide(x=w5404, y=w5397) -> (x/y=w5402:dbl[])
              n3349 = Bundle By Name(cluster=w5403, "magnitude"=w5402) -> (w5401:cluster{"f0":dbl, "df":dbl, "magnitude":dbl[]})
            }
          }
        }
        n3350 = case shown="True" w5343 {
          tunnel: w5344 -> [w5375 w5381]
          tunnel: [w5375 w5376] -> w5342
          frame False {
          }
          frame True {
            n3351 = Array Subset(array=w5381, index (row)=0 ("index"), length (row)=4 ("length"), index (col)=0 ("index"), length (col)=1 ("length")) -> (w5376:T54)
          }
        }
        n3352 = feedback-in #23(w5342) -> ()
        n3353 = Split 1D Array(array=w5356, index=2) -> (first subarray=→"FFT 1":cluster{"f0":dbl, "df":dbl, "magnitude":dbl[]}[], second subarray=→"FFT 2":cluster{"f0":dbl, "df":dbl, "magnitude":dbl[]}[])
      }
    }
    n3354 = local read "T1 calibration"() -> (w4032:T6)
    n3355 = local read "T2 calibration"() -> (w4031:T5)
    n3356 = call-poly <vilib>:"Index Waveform Array.vi"("index"=16, "waveform array"=w4006) -> ("waveform"=w4005:waveform(dbl))  [unwired: 8 in, 1 out]
    n3357 = Unbundle By Name(w4021) -> ("Y"=w4030:dbl[])
    n3358 = Unbundle By Name(w4018) -> ("Y"=w4029:dbl[])
    n3359 = Unbundle By Name(w4005) -> ("Y"=→"PSD Y Sum":dbl[])
    n3360 = call "calibrate trap data.vi"("T2 cal"=w4031, "T2"=w4029, "T1 cal"=w4032, "T1"=w4030) -> ("T2 force (pN)"=w4022:dbl[], "T2 position (nm)"=w4023:dbl[], "T1 force (pN)"=w4024:dbl[], "T1 position (nm)"=w4025:dbl[])
    n3361 = Bundle By Name(cluster=w4021, "Y"=w4025) -> (w4020:waveform(dbl))
    n3362 = Bundle By Name(cluster=w4021, "Y"=w4024) -> (w4019:waveform(dbl))
    n3363 = Bundle By Name(cluster=w4018, "Y"=w4023) -> (w4017:waveform(dbl))
    n3364 = Bundle By Name(cluster=w4018, "Y"=w4022) -> (w4016:waveform(dbl))
    n3365 = Subtract(x=w4025, y=w4023) -> (x-y=w4272:dbl[])
    n3366 = case shown="True" "Read Lateness and Rel Phase" {
      tunnel: w4102 -> [w4659 w4692]
      tunnel: w4101 -> [w4660 w4691]
      tunnel: [w4659 w4664] -> w4270
      tunnel: [w4660 w4663] -> w4269
      frame False {
      }
      frame True {
        n3367 = xnode "Read/Write Control"("FPGA VI Reference In"=w4692, "error in"=w4691) -> ("FPGA VI Reference Out"=w4666:T24, "error out"=w4665:errorcluster, "GI Relative phase"=→"GI relative phase":i16, "Relative phase"=→"Relative phase (AI1)":i16, "AI Late Counter"=→"Late Counter (AI1)":u8, "GI Late Counter"=→"GI Late Counter":u8, "MCL Late Counter"=→"MCL Late Counter":u8, "MCL Relative Phase"=→"Relative Phase (MCL)":i16, "APD Acq Relative Phase"=→"APD Acq Relative Phase":i16, "APD 1 Gate Relative Phase"=→"APD 1 Gate Relative Phase":i16, "APD 2 Gate Relative Phase"=→"APD 2 Gate Relative Phase":i16, "APD Acq Late Counter"=→"APD Acq Late Counter":u8, "APD 1 Gate Late Counter"=→"APD 1 Gate Late Counter":u8, "APD 2 Gate Late Counter"=→"APD 2 Gate Late Counter":u8, "Green FB Relative Phase"=→"Relative phase (Green FB)":i16, "GI Relative phase 2"=→"GI relative phase 2":i16, "GI Late Counter 2"=→"GI Late Counter 2":u8, "Trap Pos FIFO Timeout"=→"Trap Pos FIFO Timeout":u16, "Trap AI FIFO Timeout"=→"Trap AI FIFO Timeout":u16, "RI Late Counter"=→"RI Late Counter":u8, "RI Relative phase"=→"RI relative phase":i16, "Green Late Counter"=→"Green AI Late Counter":u8, "BI Late Counter (AO)"=→"Late Counter (BI AO)":u8, "Blue Late Counter (D)"=→"Late Counter (BI DO)":u8, "BI Relative phase (AO)"=→"Relative phase (BI AO)":i16, "BI Relative phase (D)"=→"Relative phase (BI DO)":i16)
        n3368 = xnode "Read/Write Control"("FPGA VI Reference In"=w4666, "error in"=w4665) -> ("FPGA VI Reference Out"=w4664:T24, "error out"=w4663:errorcluster, "APD 3 Gate Late Counter"=→"APD 3 Gate Late Counter":u8, "APD 3 Gate Relative Phase"=→"APD 3 Gate Relative Phase":i16)
      }
    }
    n3369 = Negate(x=w4272) -> (-x=w4085:dbl[])
    n3370 = Subtract(x=w4085, y="Offset (nm)") -> (x-y=w4246:dbl[])
    n3371 = case "Choose calibrated display" shown="2" "Calibration" {
      tunnel: w4021 -> [w4694 _ _]
      tunnel: w4018 -> [w4693 _ _]
      tunnel: [w4694 w4696 w4698] -> w4285
      tunnel: [w4693 w4695 w4697] -> w4284
      tunnel: w4020 -> [_ w4696 _]
      tunnel: w4019 -> [_ _ w4698]
      tunnel: w4017 -> [_ w4695 _]
      tunnel: w4016 -> [_ _ w4697]
      frame 0, Default {
      }
      frame 1 {
      }
      frame 2 {
      }
    }
    n3372 = Bundle By Name(cluster=w4021, "Y"=w4246) -> (w4015:waveform(dbl))
    "Bead Separation" <- w4015
    n3373 = feedback #24(w4246) -> (w4245:dbl[])
    n3374 = Build Array (concatenate)(w4246, w4245) -> (w4027:dbl[])
    n3375 = Split 1D Array(array=w4027, index=w4145) -> (first subarray=w4028:dbl[])  [unwired: 1 out]
    n3376 = feedback-in #24(w4028) -> ()
    n3377 = Build Array(w4021, w4020, w4019, w4018, w4017, w4016, w4015) -> (w4014:waveform(dbl)[])
    n3378 = Not(x="Trap Trig. Fl.") -> (.not. x?=w4121:bool)
    n3379 = Unbundle By Name(w4285) -> ("Y"=w4086:dbl[])
    n3380 = Unbundle By Name(w4284) -> ("Y"=w4247:dbl[])
    n3381 = call-poly <vilib>:"Mean.vi"("X"=w4028) -> ("mean"=w4242:dbl)  [unwired: 1 out]
    "Bead Mean (nm)" <- w4242
    n3382 = Multiply(x=w4284, y=-1.0) -> (x*y=w4274:waveform(dbl))
    n3383 = call-poly <vilib>:"Mean.vi"("X"=w4086) -> ("mean"=w4089:dbl)  [unwired: 1 out]
    "T1 X" <- w4089
    n3384 = call-poly <vilib>:"Mean.vi"("X"=w4247) -> ("mean"=w4088:dbl)  [unwired: 1 out]
    "T2 X" <- w4088
    n3385 = Build Array(w4285, w4274) -> (→"Force":waveform(dbl)[])
    n3386 = Subtract(x=w4028, y=w4242) -> (x-y=w4241:dbl[])
    n3387 = Square(x=w4241) -> (x^2=w4240:dbl[])
    n3388 = Negate(x=w4247) -> (-x=w4039:dbl[])
    n3389 = call-poly <vilib>:"Mean.vi"("X"=w4240) -> ("mean"=w4239:dbl)  [unwired: 1 out]
    n3390 = Negate(x=w4088) -> (-x=w4087:dbl)
    n3391 = Square Root(x=w4239) -> (sqrt(x)=w4238:dbl)
    n3392 = Add(x=w4086, y=w4039) -> (x+y=w4248:dbl[])
    n3393 = Add(x=w4089, y=w4087) -> (x+y=w4279:dbl)
    n3394 = Multiply(x=10.0, y=w4238) -> (x*y=→"RMS (Ang)":dbl)
    n3395 = Divide(x=w4248, y=2.0) -> (x/y=w4042:dbl[])
    n3396 = Subtract(x=w4089, y=w4087) -> (x-y=→"Difference":dbl)
    n3397 = Select(t=w4039, s="Only check fixed trap T2", f=w4042) -> (s? t:f=→"Vec Mean of T1 T2":dbl[])
    n3398 = Divide(x=w4279, y=2.0) -> (x/y=w4250:dbl)
    "Mean" <- w4250
    n3399 = feedback-in #25("Trap Trig. Fl.") -> ()
    n3400 = feedback #25("Trap Trig. Fl.") -> (w4119:bool)
    n3401 = And(x=w4121, y=w4119) -> (x .and. y?=w4120:bool)
    n3402 = case "If have just turned off triggering" shown="True" w4120 {
      tunnel: w4102 -> [_ w4494]
      tunnel: w4101 -> [_ w4493]
      frame False {
      }
      frame True {
        w4492 = FALSE ("FPGA Trap Trig")
        n3403 = xnode "Read/Write Control"("FPGA VI Reference In"=w4494, "error in"=w4493, "FPGA Trap Trig"=w4492) -> ("FPGA VI Reference Out"=w4491:T24, "error out"=w4490:errorcluster)
        n3404 = xnode "Read/Write Control"("FPGA VI Reference In"=w4491, "error in"=w4490, "TTrig?"=w4492) -> ()  [unwired: 2 out]
        n3405 = local write "Initializing"(FALSE ("Initializing")) -> ()
        n3406 = local write "Triggered"(FALSE ("Triggered")) -> ()
        n3407 = local write "Waiting"(FALSE ("Waiting")) -> ()
      }
    }
    n3408 = Not(x=w4119) -> (.not. x?=w4132:bool)
    n3409 = And(x="Trap Trig. Fl.", y=w4132) -> (x .and. y?=w4129:bool)
    n3410 = Or(x=w4129, y="Reinitialize") -> (x .or. y?=w4115:bool)
    n3411 = feedback #26(w4125) -> (w4130:string)
    n3412 = Select(t=w4125, s=w4129, f=w4130) -> (s? t:f=w4124:string)
    n3413 = Select(t=w4125, s="Reinitialize", f=w4124) -> (s? t:f=w4123:string)
    n3414 = local read "Tether"() -> (w4251:bool)
    n3415 = feedback #27(0) -> (w4127:i32)
    n3416 = case "For determining if there is a tether still" shown="True" w4251 {
      tunnel: w4250 -> [_ w4618]
      frame False {
      }
      frame True {
        n3417 = Greater?(x="Lost Tether Alarm Threshold (pN)", y=w4618) -> (0:w4616:bool)
        n3418 = case shown="True" w4616 {
          frame False {
          }
          frame True {
            w4619 = FALSE ("Value (Signaling)")